vi "VP_RT_standard.vi"() -> ()   [LabVIEW 2015] (continued)
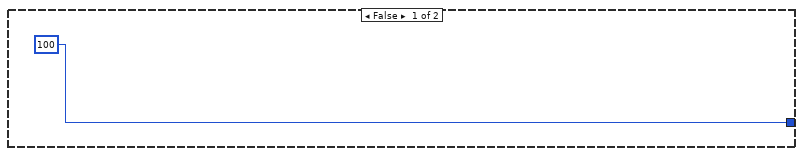
[diagram p2: hidden frame]
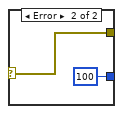
[diagram p3: hidden frame]
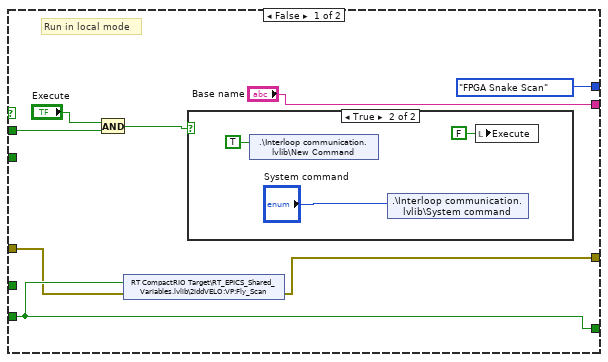
[diagram p4: hidden frame]
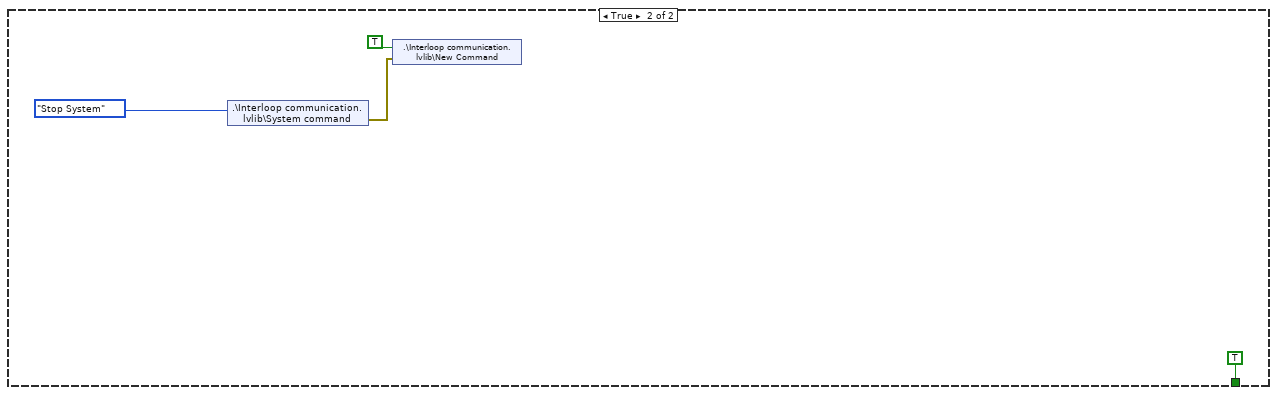
[diagram p7: hidden frame]
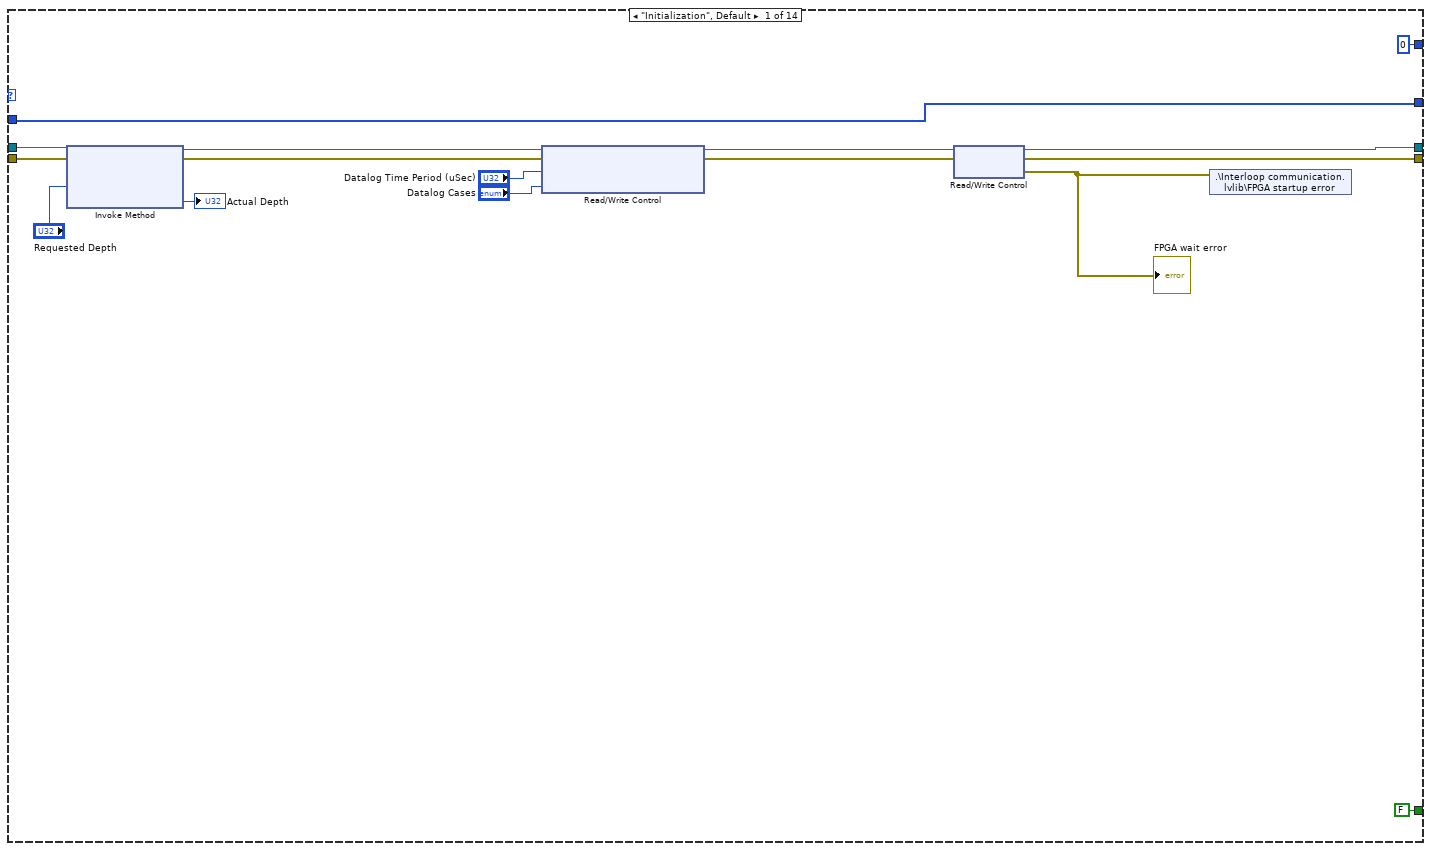
[diagram p8: hidden frame]
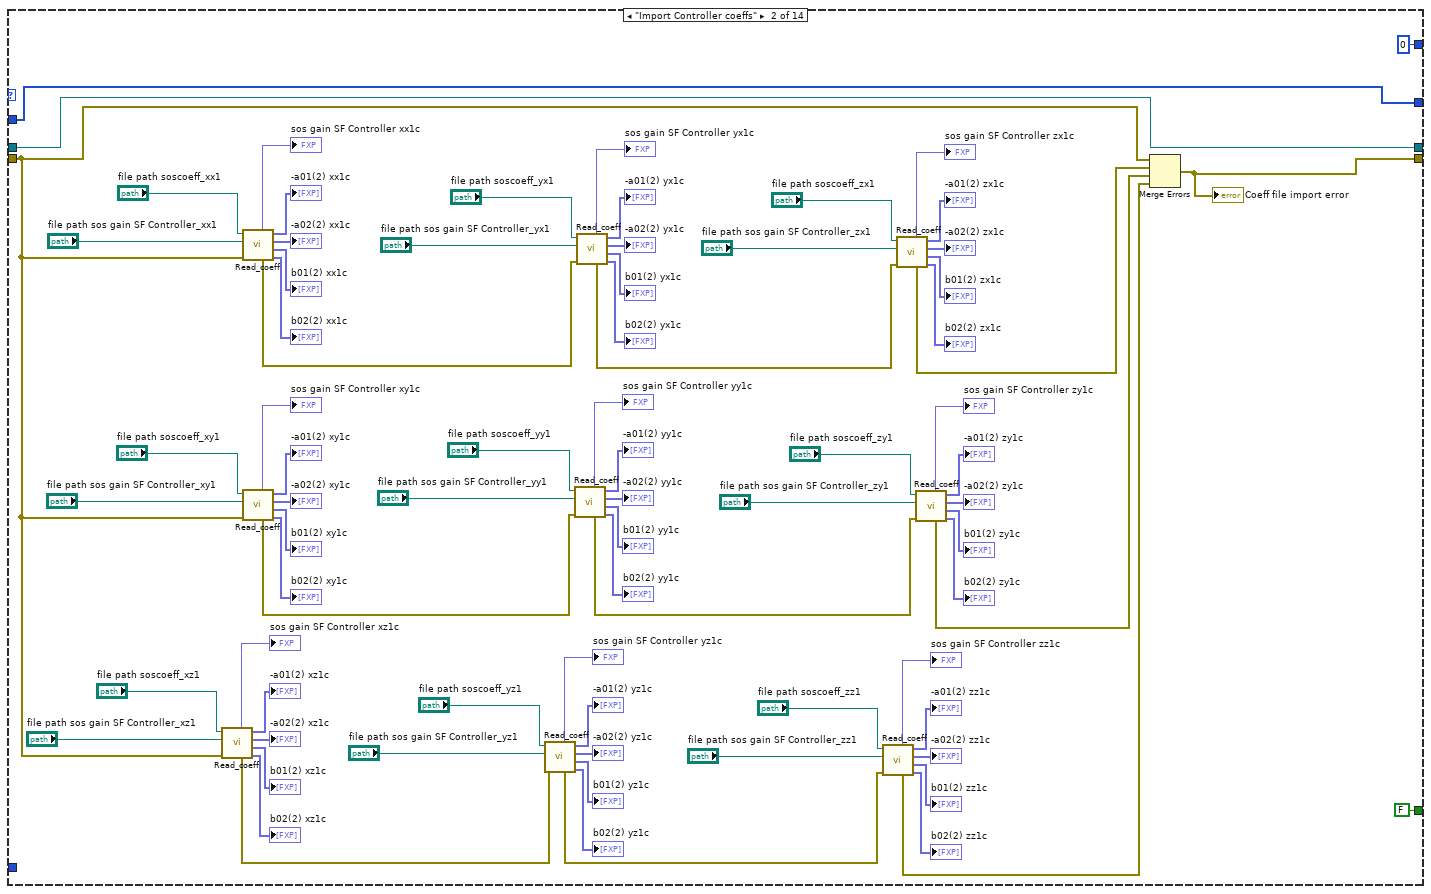
[diagram p9: hidden frame]
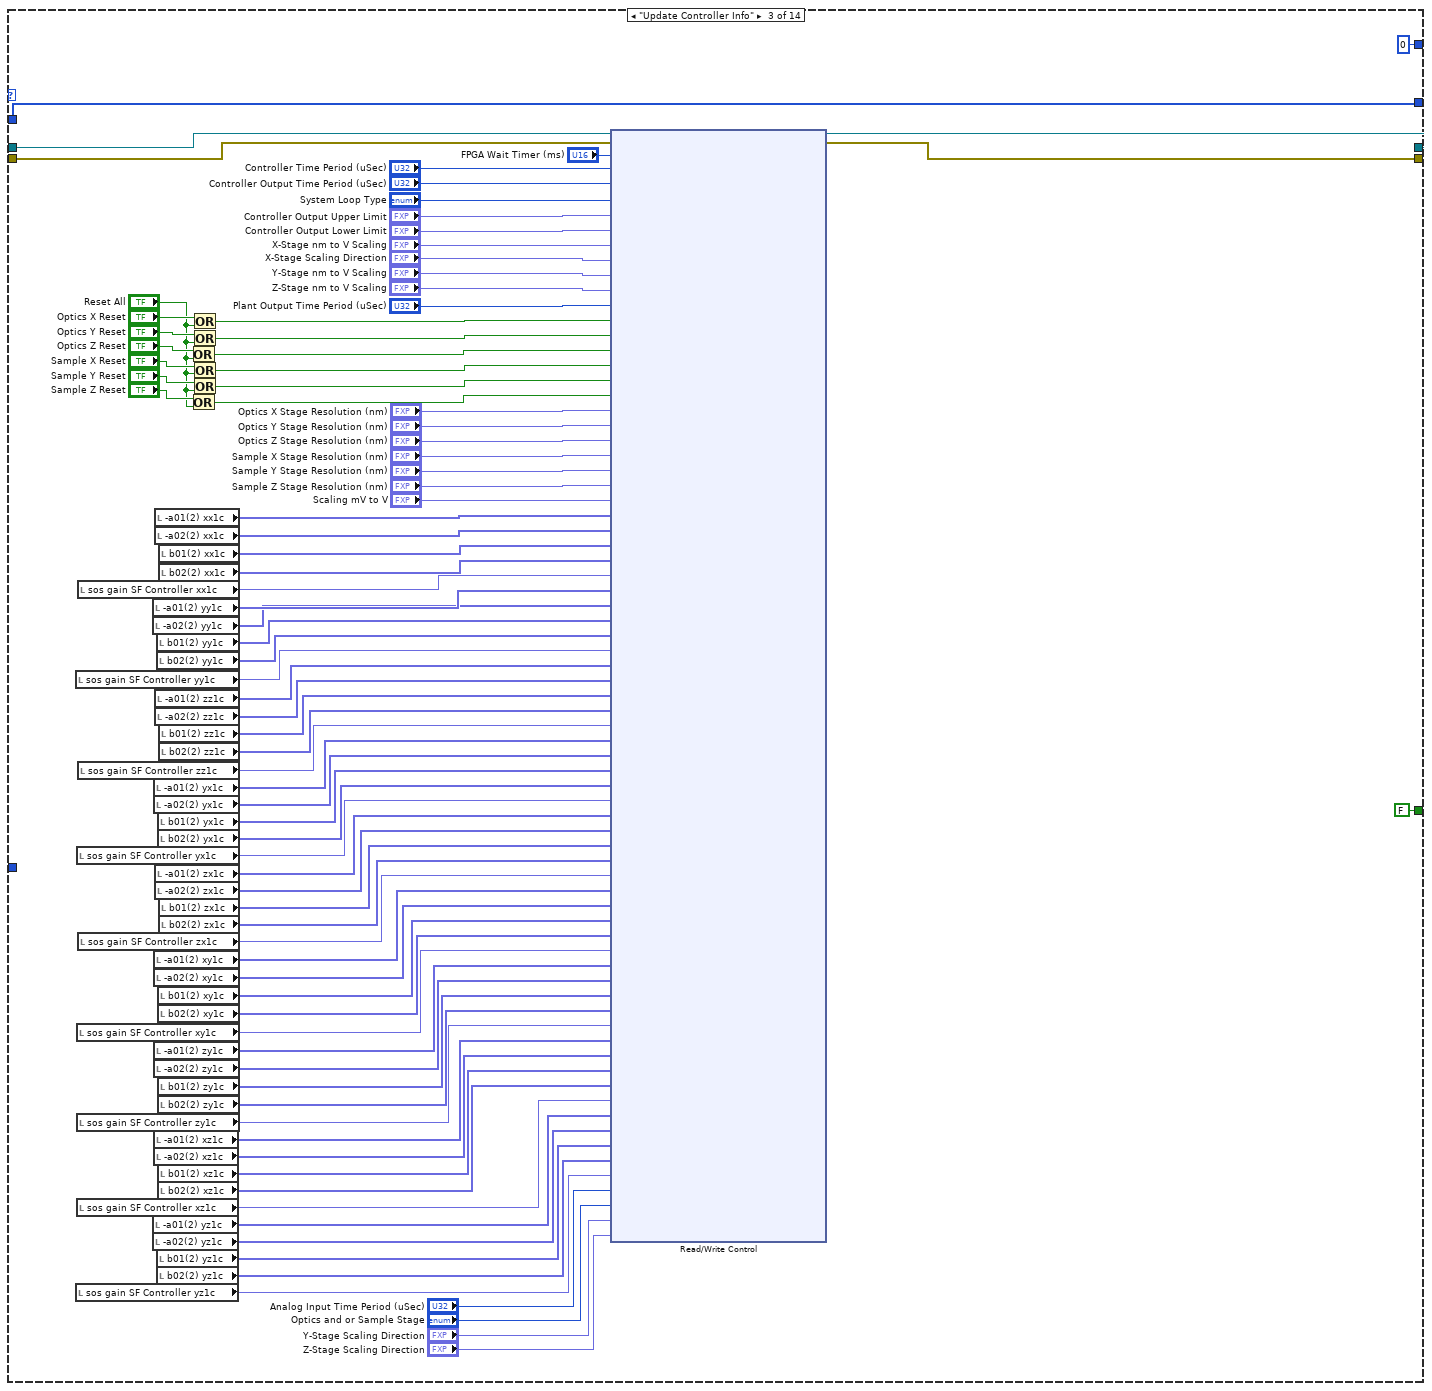
[diagram p10: hidden frame]
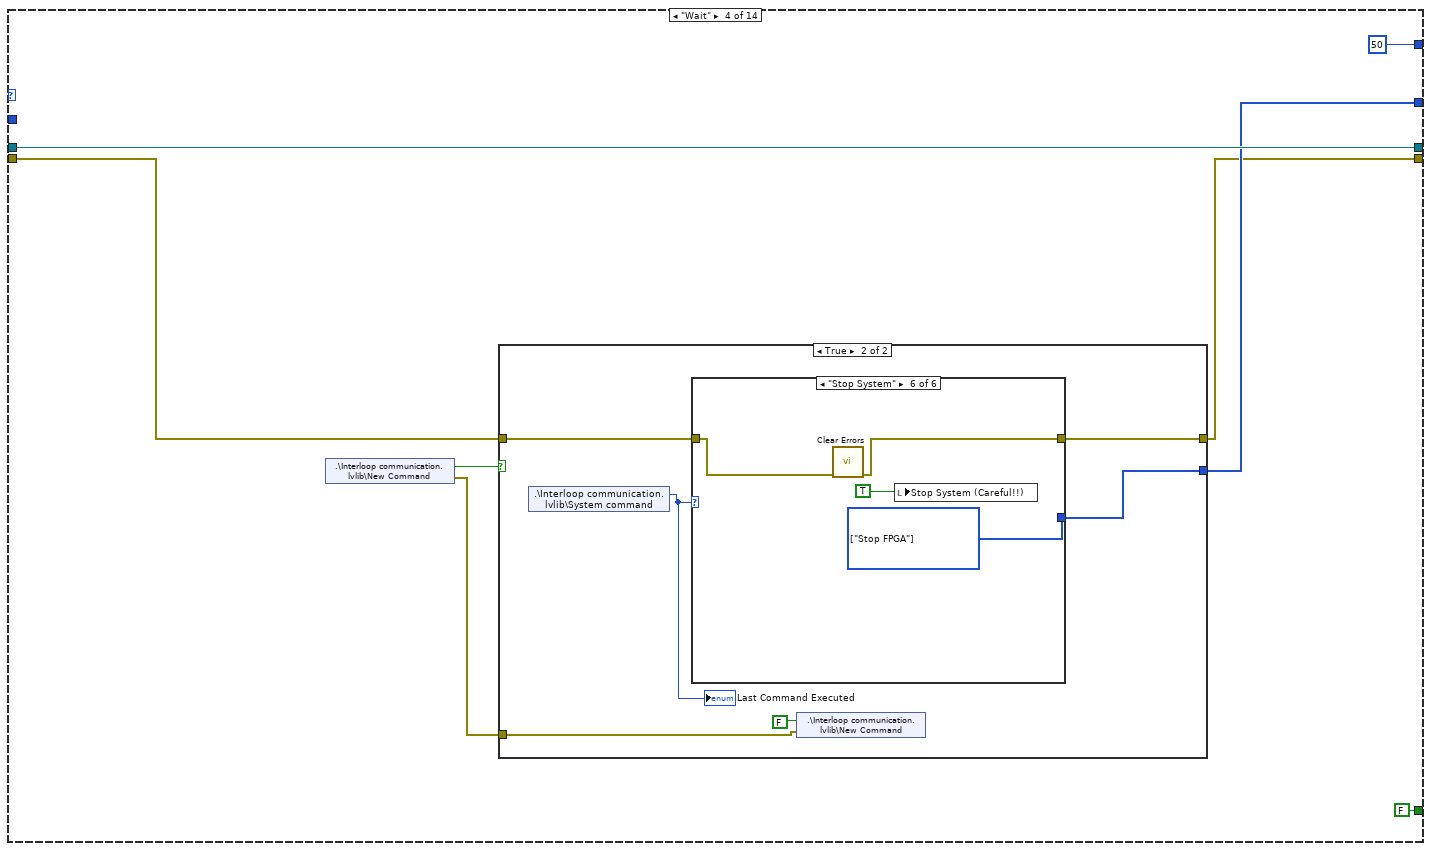
[diagram p11: hidden frame]
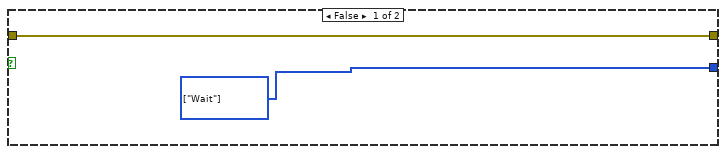
[diagram p12: hidden frame]
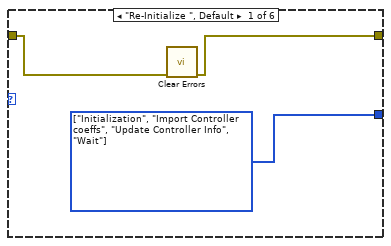
[diagram p13: hidden frame]
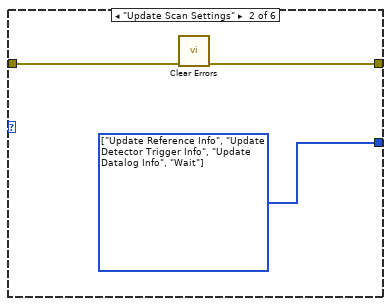
[diagram p14: hidden frame]
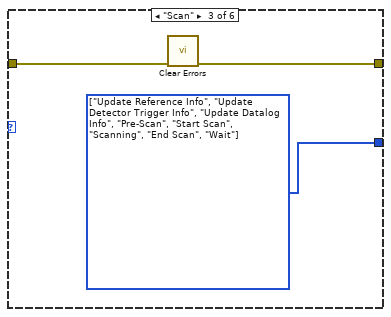
[diagram p15: hidden frame]
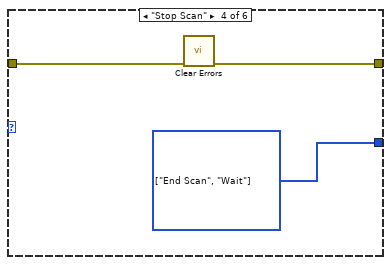
[diagram p16: hidden frame]
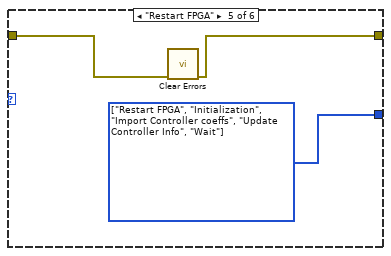
[diagram p17: hidden frame]
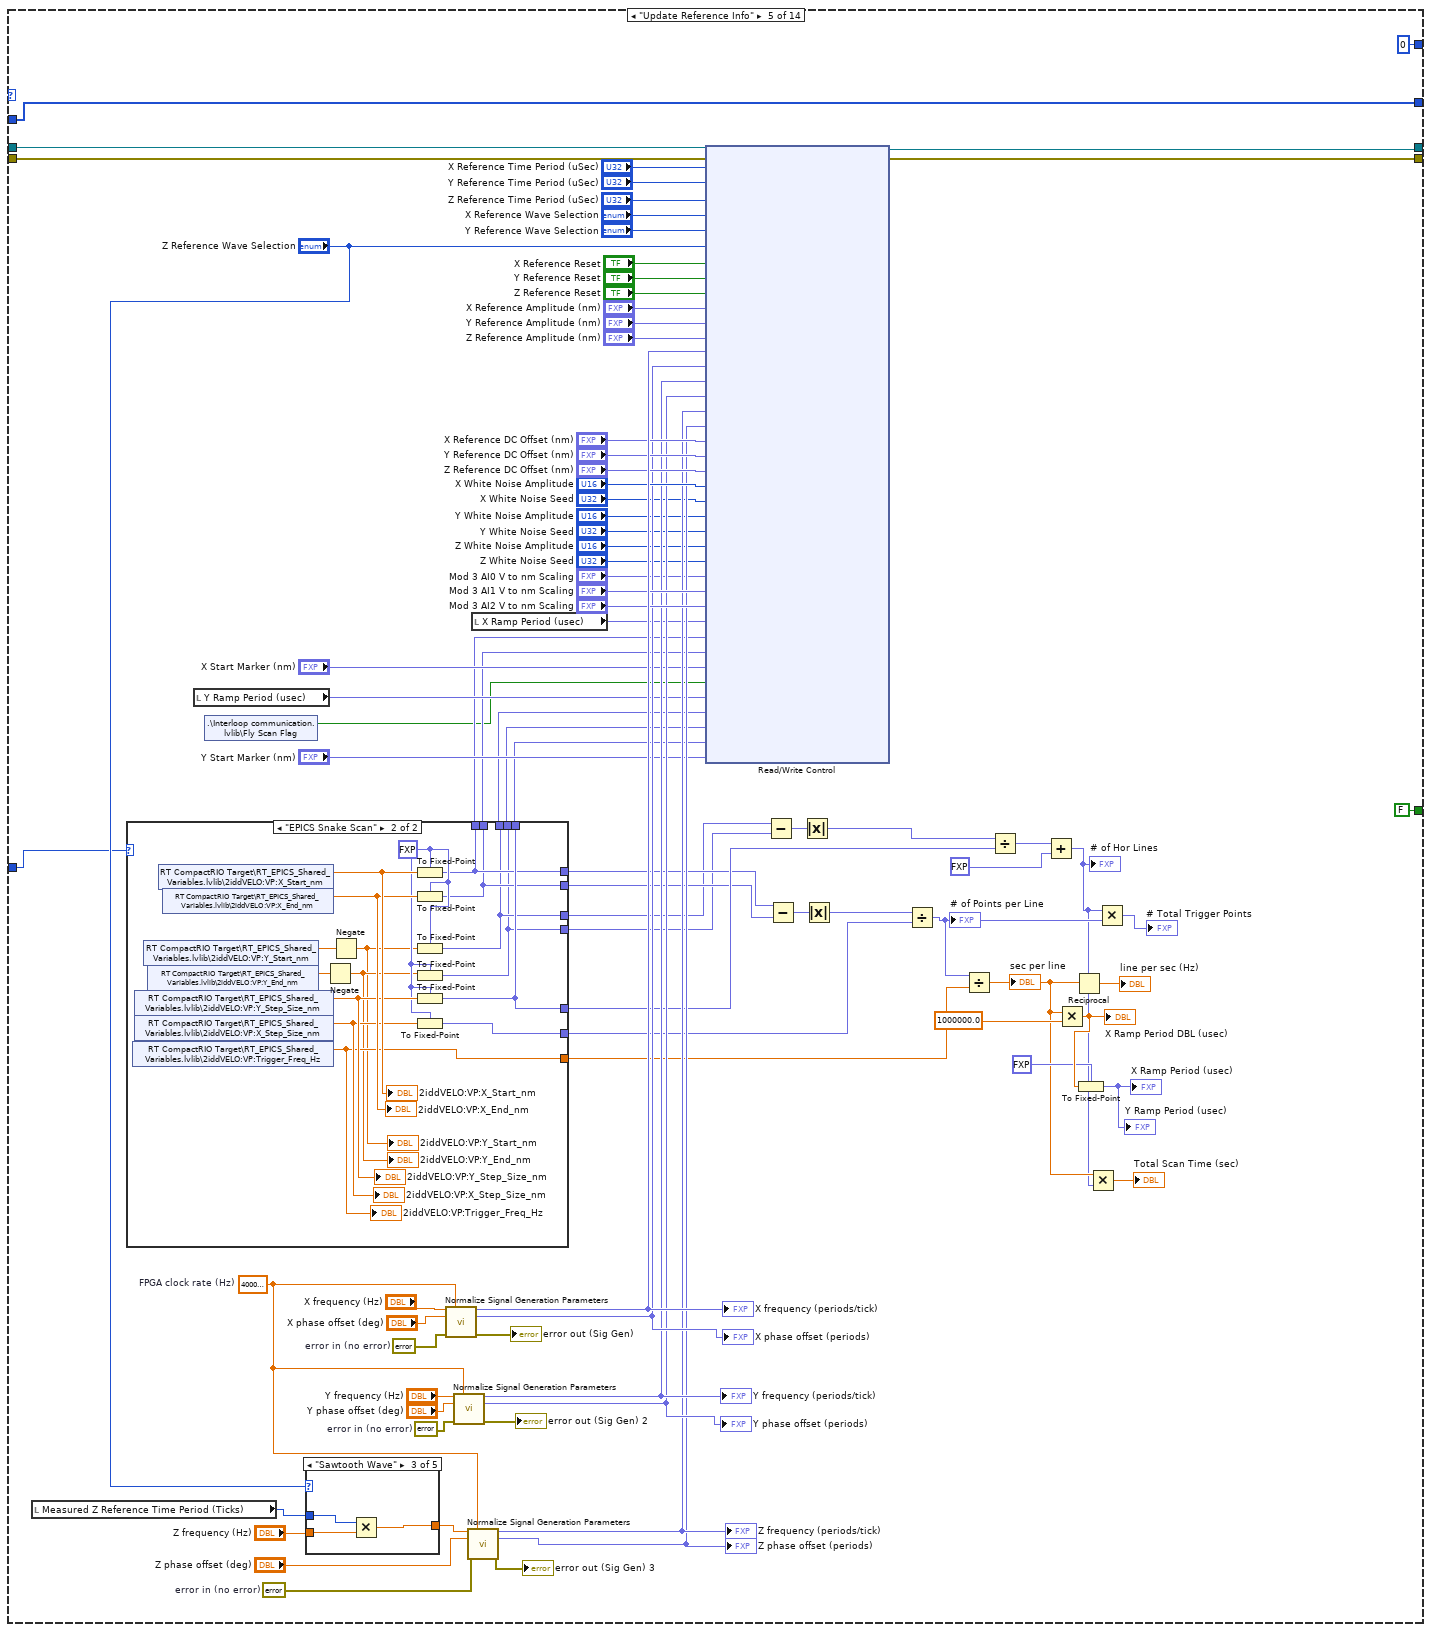
[diagram p18: hidden frame]
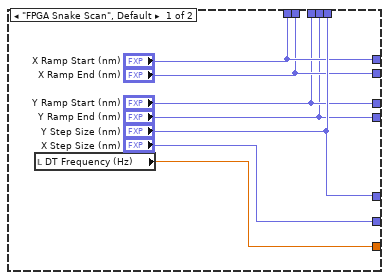
[diagram p19: hidden frame]
        n233 = Bundle("Array"=w587, "Array"=w586) -> (→"XY actual":cluster{"Array":dbl[], "Array":dbl[]})  [unwired: 1 in]
        n234 = Merge Errors(w579, w573) -> (w578:errorcluster)
      }
      frame "End Scan" {
        n235 = xnode "Invoke Method"("FPGA VI Reference In"=w616, "error in"=w614) -> ("FPGA VI Reference Out"=w615:refnum<k20>, "error out"=w613:errorcluster)
        n236 = xnode "Read/Write Control"("FPGA VI Reference In"=w615, "error in"=w613, "stop case"=TRUE ("New FPGA command")) -> ("FPGA VI Reference Out"=w619:refnum<k20>, "error out"=w618:errorcluster)
        n237 = shared-variable "RT CompactRIO Target\\RT_EPICS_Shared_Variables.lvlib\\2iddVELO:VP:Scanning"(FALSE ("2iddVELO:VP:Fly_Scanning")) -> ()  [unwired: 1 in, 1 out]
        n238 = call "Data_Write.vi"("error initialize"=w618, "Command List"=Data_Write_Control."Close") -> ("error out"=w612:errorcluster)  [unwired: 6 in, 1 out]
        n239 = case shown="No Error" w612 {
          tunnel: w612 -> [w630 w631]
          tunnel: [w629 w631] -> w622
          frame No Error {
            n240 = local read "Output filename"() -> (w626:string)
            n241 = local read "Output path"() -> (w627:path)
            n242 = Path To String(path=w627) -> (string=w625:string)
            n243 = shared-variable "RT CompactRIO Target\\RT_EPICS_Shared_Variables.lvlib\\2iddVELO:VP:Last_Filename"(w626, error in=w630) -> (error out=w628:errorcluster)
            n244 = shared-variable "RT CompactRIO Target\\RT_EPICS_Shared_Variables.lvlib\\2iddVELO:VP:cRIO_Dir"(w625, error in=w628) -> (error out=w629:errorcluster)
          }
          frame Error {
          }
        }
      }
      frame "Restart FPGA" {
        n245 = call <vilib>:"Clear Errors.vi"("error in (no error)"=w637) -> ("error out"=w638:errorcluster)  [unwired: 5 in, 1 out]
        n246 = xnode "Invoke Method"("FPGA VI Reference In"=w643, "error in"=w638) -> ("FPGA VI Reference Out"=w642:refnum<k20>, "error out"=w641:errorcluster)
        n247 = xnode "Read/Write Control"("FPGA VI Reference In"=w642, "error in"=w641, "stop case"=TRUE) -> ("FPGA VI Reference Out"=w636:refnum<k20>, "error out"=w635:errorcluster)
        n248 = xnode "Invoke Method"("FPGA VI Reference In"=w636, "error in"=w635) -> ("FPGA VI Reference Out"=w634:refnum<k20>, "error out"=w633:errorcluster)
      }
      frame "Stop FPGA" {
        w651 = T10[] [enum."Stop FPGA"] items=["Initialization", "Import Controller coeffs", "Update Controller Info", "Wait", "Update Reference Info", "Update Detector Trigger Info", "Update Datalog Info", "Check FPGA Status", "Pre-Scan", "Start Scan", "Scanning", "End Scan", "Restart FPGA", "Stop FPGA"] ("Reduced Array of States")
        w650 = TRUE ("stop case")
        n249 = xnode "Invoke Method"("FPGA VI Reference In"=w658, "error in"=w657) -> ("FPGA VI Reference Out"=w656:refnum<k20>, "error out"=w655:errorcluster)
        n250 = xnode "Read/Write Control"("FPGA VI Reference In"=w656, "error in"=w655, "stop case"=w650, "New FPGA command"=w650, "FPGA command"=enum16{"Start Scan", "Shutdown"}."Shutdown") -> ("FPGA VI Reference Out"=w654:refnum<k20>, "error out"=w647:errorcluster)
        n251 = xnode "Invoke Method"("FPGA VI Reference In"=w654, "error in"=w647) -> ("FPGA VI Reference Out"=w648:refnum<k20>, "error out"=w646:errorcluster)
        n252 = xnode "Close FPGA VI Reference"("FPGA VI Reference In"=w648, "error in"=w646) -> ("error out"=w653:errorcluster)
      }
    }
    "Main Loop error" <- w82
    n253 = shared-variable ".\\Interloop communication.lvlib\\Main Loop Error"(w82) -> ()  [unwired: 1 in, 1 out]
    n254 = node-c288(w77) -> ()  [unwired: 1 out]
    n255 = call "State Control.vi"("Stop"=FALSE, "Array of States"=w84, "Error Input"=w82) -> ("Next State"=w74:T10, "Reduced Array of States"=w78:T10[])  [unwired: 5 in]
    "RT Main Loop State" <- w71
    "Main Loop Iterations" <- w80
    "Reduced Array of States" <- w79
  }
  n256 = while {
    tunnel: w2 -> [w667]
    tunnel: w1 -> [w666]
    i -> [w664]
    stop <- w665 stop-if-true
    # "Readback loop"
    n257 = local read "RT Main Loop State"() -> (w670:T10)
    n258 = Not Equal?(x=w670, y=State_Enum."Initialization") -> (x != y?=w668:bool)
    n259 = case shown="True" w668 {
      tunnel: w667 -> [_ w678]
      tunnel: w666 -> [_ w676]
      tunnel: [u32 100 ("milliseconds to wait") "Readback Loop time between iterations (ms)"] -> w663
      frame False {
      }
      frame True {
        w717 = 40000000.0  # FPGA Clock Rate (Hz)
        w736 = 40000000.0  # FPGA Clock Rate (Hz)
        w753 = 40000000.0  # FPGA Clock Rate (Hz)
        n260 = xnode "Read/Write Control"("FPGA VI Reference In"=w678, "error in"=w676) -> ("FPGA VI Reference Out"=w677:refnum<k20>, "error out"=w675:errorcluster, "FPGA state"=w674:T9, "Fly scan completed"=→"Fly Scan Complete":bool)
        "FPGA state" <- w674
        n261 = Format Into String(format string="%s", w674) -> (resulting string=w673:string)  [unwired: 2 in, 1 out]
        n262 = xnode "Read/Write Control"("FPGA VI Reference In"=w677, "error in"=w675) -> ("error out"=w684:errorcluster, "Measured Datalog Time Period (Ticks)"=w711:u32, "Measured Counter Time Period (Ticks)"=w716:u32, "Mod4/DIO0"=→"Mod4/DIO0":bool, "Mod4/DIO1"=→"Mod4/DIO1":bool, "Mod4/DIO2"=→"Mod4/DIO2":bool, "Mod4/DIO3"=→"Mod4/DIO3":bool, "Mod5/DIO0"=→"Mod5/DIO0":bool, "Mod5/DIO1"=→"Mod5/DIO1":bool, "Mod5/DIO2"=→"Mod5/DIO2":bool, "Mod5/DIO3"=→"Mod5/DIO3":bool, "Mod6/DIO0"=→"Mod6/DIO0":bool, "Mod6/DIO1"=→"Mod6/DIO1":bool, "Mod6/DIO2"=→"Mod6/DIO2":bool, "Mod6/DIO3"=→"Mod6/DIO3":bool, "32 bit Count Optics X"=→"32 bit Count Optics X":i32, "32 bit Count Optics  Y"=→"32 bit Count Optics  Y":i32, "32 bit Count Optics  Z"=→"32 bit Count Optics  Z":i32, "32 bit Count Sample X"=→"32 bit Count Sample X":i32, "32 bit Count Sample  Y"=→"32 bit Count Sample  Y":i32, "32 bit Count Sample  Z"=→"32 bit Count Sample  Z":i32, "Optics X Stage Displacement (nm)"=→"Optics X Stage Displacement (nm)":fxp<+/-,58,25>, "Optics Y Stage Displacement (nm)"=→"Optics Y Stage Displacement (nm)":fxp<+/-,58,25>, "Optics Z Stage Displacement (nm)"=→"Optics Z Stage Displacement (nm)":fxp<+/-,58,25>, "Sample X Stage Displacement (nm)"=→"Sample X Stage Displacement (nm)":fxp<+/-,58,25>, "Sample Y Stage Displacement (nm)"=→"Sample Y Stage Displacement (nm)":fxp<+/-,58,25>, "Sample Z Stage Displacement (nm)"=→"Sample Z Stage Displacement (nm)":fxp<+/-,58,25>)  [unwired: 1 out]
        "Measured Datalog Time Period (Ticks)" <- w711
        "Measured Counter Time Period (Ticks)" <- w716
        n263 = xnode "Read/Write Control"("FPGA VI Reference In"=w677, "error in"=w675) -> ("error out"=w683:errorcluster, "Measured Detector Trigger Time Period (Ticks)"=→"Measured Detector Trigger Time Period (Ticks)":u32, "Measured Trigger Gen Time Period (Ticks)"=→"Measured Trigger Gen Time Period (Ticks)":u32, "Detector Trigger (V)"=→"Detector Trigger (V)":fxp<+/-,20,5>, "Detector Trigger In Range?"=→"Detector Trigger In Range?":bool, "Measured Data Trigger Time Period (Ticks)"=→"Measured Data Trigger Time Period (Ticks)":u32, "Trigger for Data"=→"Trigger for Data":fxp<+/-,58,25>)  [unwired: 1 out]
        n264 = xnode "Read/Write Control"("FPGA VI Reference In"=w677, "error in"=w675) -> ("error out"=w681:errorcluster, "PI X-Stage Input (V)"=→"PI X-Stage Input (V)":fxp<+/-,20,5>, "PI Y-Stage Input (V)"=→"PI Y-Stage Input (V)":fxp<+/-,20,5>, "PI Z-Stage Input (V)"=→"PI Z-Stage Input (V)":fxp<+/-,20,5>, "X-Stage Input In Range?"=→"X-Stage Input In Range?":bool, "Y-Stage Input In Range?"=→"Y-Stage Input In Range?":bool, "Z-Stage Input In Range?"=→"Z-Stage Input In Range?":bool, "Measured Controller Time Period (Ticks)"=w757:u32, "Measured Controller Output Time Period (Ticks)"=w756:u32, "Measured Plant Output Time Period (Ticks)"=w755:u32, "Measured Analog Input Time Period (Ticks)"=w754:u32)  [unwired: 1 out]
        "Measured Controller Time Period (Ticks)" <- w757
        "Measured Controller Output Time Period (Ticks)" <- w756
        "Measured Plant Output Time Period (Ticks)" <- w755
        "Measured Analog Input Time Period (Ticks)" <- w754
        n265 = xnode "Read/Write Control"("FPGA VI Reference In"=w677, "error in"=w675) -> ("error out"=w682:errorcluster, "X Stage Reference (nm)"=→"X Stage Reference (nm)":fxp<+/-,58,25>, "Y Stage Reference (nm)"=→"Y Stage Reference (nm)":fxp<+/-,58,25>, "Z Stage Reference (nm)"=→"Z Stage Reference (nm)":fxp<+/-,58,25>, "Measured X Reference Time Period (Ticks)"=w738:u32, "Measured Y Reference Time Period (Ticks)"=w737:u32, "Measured Z Reference Time Period (Ticks)"=w729:u32, "Fly Scan Running"=→"Fly Scan Running":bool, "Continue Run"=→"Continue Run":bool)  [unwired: 1 out]
        "Measured X Reference Time Period (Ticks)" <- w738
        "Measured Y Reference Time Period (Ticks)" <- w737
        "Measured Z Reference Time Period (Ticks)" <- w729
        n266 = shared-variable "RT CompactRIO Target\\RT_EPICS_Shared_Variables.lvlib\\2iddVELO:VP:FPGA_State"(w673) -> ()  [unwired: 1 in, 1 out]
        n267 = call "Convert Measured Rate.vi"("FPGA Clock Rate (Hz)"=w736, "Measured Reference Time Period (Ticks)"=w729) -> ("Measured Reference Loop Rate (kHz)"=→"Measured Z Reference Loop Rate (kHz)":dbl, "Measured Reference Loop Period (s)"=→"Measured Z Reference Loop Rate (secs)":dbl)
        n268 = call "Convert Measured Rate.vi"("FPGA Clock Rate (Hz)"=w736, "Measured Reference Time Period (Ticks)"=w737) -> ("Measured Reference Loop Rate (kHz)"=→"Measured Y Reference Loop Rate (kHz)":dbl, "Measured Reference Loop Period (s)"=→"Measured Y Reference Loop Rate (secs)":dbl)
        n269 = call "Convert Measured Rate.vi"("FPGA Clock Rate (Hz)"=w717, "Measured Reference Time Period (Ticks)"=w716) -> ("Measured Reference Loop Rate (kHz)"=w714:dbl, "Measured Reference Loop Period (s)"=→"Measured Counter Loop Rate (secs)":dbl)
        n270 = call "Convert Measured Rate.vi"("FPGA Clock Rate (Hz)"=w736, "Measured Reference Time Period (Ticks)"=w738) -> ("Measured Reference Loop Rate (kHz)"=→"Measured X Reference Loop Rate (kHz)":dbl, "Measured Reference Loop Period (s)"=→"Measured X Reference Loop Rate (secs)":dbl)
        n271 = call "Convert Measured Rate.vi"("FPGA Clock Rate (Hz)"=w717, "Measured Reference Time Period (Ticks)"=w711) -> ("Measured Reference Loop Rate (kHz)"=→"Measured Datalog Loop Rate (kHz)":dbl, "Measured Reference Loop Period (s)"=→"Measured Datalog Loop Rate (secs)":dbl)
        n272 = call "Convert Measured Rate.vi"("FPGA Clock Rate (Hz)"=w753, "Measured Reference Time Period (Ticks)"=w757) -> ("Measured Reference Loop Rate (kHz)"=→"Measured Controller Loop Rate (kHz)":dbl, "Measured Reference Loop Period (s)"=→"Measured Controller Loop Rate (secs)":dbl)
        n273 = call "Convert Measured Rate.vi"("FPGA Clock Rate (Hz)"=w753, "Measured Reference Time Period (Ticks)"=w756) -> ("Measured Reference Loop Rate (kHz)"=→"Measured Controller Output Loop Rate (kHz)":dbl, "Measured Reference Loop Period (s)"=→"Measured Controller Output Loop Rate (secs)":dbl)
        n274 = call "Convert Measured Rate.vi"("FPGA Clock Rate (Hz)"=w753, "Measured Reference Time Period (Ticks)"=w755) -> ("Measured Reference Loop Rate (kHz)"=→"Measured Plant Output Loop Rate (kHz)":dbl, "Measured Reference Loop Period (s)"=→"Measured Plant Output Loop Rate (secs)":dbl)
        n275 = call "Convert Measured Rate.vi"("FPGA Clock Rate (Hz)"=w753, "Measured Reference Time Period (Ticks)"=w754) -> ("Measured Reference Loop Rate (kHz)"=→"Measured Analog Input Loop Rate (kHz)":dbl, "Measured Reference Loop Period (s)"=→"Measured Analog Input Loop Rate (secs)":dbl)
        n276 = Divide(x=w714, y=1000.0) -> (x/y=→"Measured Counter Loop Rate (MHz)":dbl)
        n277 = Merge Errors(w681, w682, w683, w684) -> (w680:errorcluster)
        "Readback error" <- w680
        n278 = shared-variable ".\\Interloop communication.lvlib\\Readback Loop Error"(w680) -> ()  [unwired: 1 in, 1 out]
      }
    }
    n279 = local read "Stop System (Careful!!)"() -> (w665:bool)
    n280 = Wait (ms)(milliseconds to wait=w663) -> ()  [unwired: 1 out]
    "Readback loop Iterations" <- w664
  }
  n281 = while {
    shift-right: [w771] -> _
    shift-left: TRUE -> [w772]
    i -> [w759]
    stop <- w764 stop-if-true
    # "Heartbeat Loop"
    n282 = shared-variable ".\\Interloop communication.lvlib\\Command Loop Error"() -> (w766:errorcluster)  [unwired: 1 in, 1 out]
    n283 = shared-variable ".\\Interloop communication.lvlib\\FPGA startup error"() -> (w762:errorcluster)  [unwired: 1 in, 1 out]
    n284 = Not(x=w772) -> (.not. x?=w771:bool)
    "Heartbeat" <- w771
    n285 = shared-variable ".\\Interloop communication.lvlib\\Readback Loop Error"() -> (w765:errorcluster)  [unwired: 1 in, 1 out]
    n286 = shared-variable ".\\Interloop communication.lvlib\\Main Loop Error"() -> (w770:errorcluster)  [unwired: 1 in, 1 out]
    n287 = call <vilib>:"RT LEDs.vi"("State"=3, "LED Num"=0) -> ("error out"=w763:errorcluster)  [unwired: 4 in, 1 out]
    n288 = Merge Errors(w763, w766, w762, w770, w765) -> (w767:errorcluster)
    n289 = case shown="No Error" w767 {
      selector: w767 -> [w773 w775]
      tunnel: [u32 500 ("millisecond multiple") u32 100 ("millisecond multiple")] -> w769
      tunnel: [w773 w775] -> w768
      frame No Error {
      }
      frame Error {
      }
    }
    "RT error" <- w768
    n290 = local read "Stop System (Careful!!)"() -> (w764:bool)
    n291 = Wait Until Next ms Multiple(millisecond multiple=w769) -> ()  [unwired: 1 out]
    "Heartbeat Loop Iterations" <- w759
  }
  n292 = while {
    stop <- w780 stop-if-true
    n293 = shared-variable "RT CompactRIO Target\\RT_EPICS_Shared_Variables.lvlib\\2iddVELO:VP:cRIO_Command"() -> (→"2iddVELO:VP:cRIO_Command":string)  [unwired: 1 in, 1 out]
    n294 = shared-variable "RT CompactRIO Target\\RT_EPICS_Shared_Variables.lvlib\\2iddVELO:VP:Controller_Type"() -> (→"2iddVELO:VP:Controller_Type":string)  [unwired: 1 in, 1 out]
    n295 = shared-variable "RT CompactRIO Target\\RT_EPICS_Shared_Variables.lvlib\\2iddVELO:VP:Scan_Type"() -> (→"2iddVELO:VP:Scan_Type":string)  [unwired: 1 in, 1 out]
    n296 = local read "Stop System (Careful!!)"() -> (w780:bool)
    n297 = Wait Until Next ms Multiple(millisecond multiple=u32 250) -> ()  [unwired: 1 out]
  }
  n298 = node-c288(w8) -> (→"Timed Loop (end error)":errorcluster, →"Iteration Duration RT Timed-Loop":i64)
